vi "FlexMag - 23-03-2023.vi"() -> ()   [LabVIEW 2018] (continued)
                    n16430 = local read "abort ch3"() -> (w21515:bool)
                    n16431 = case shown="False" w21515 {
                      frame False {
                        n16432 = while {
                          i -> [w21518]
                          stop <- w21521 stop-if-true
                          n16433 = Greater Or Equal?(x=w21518, y=100) -> (x >= y?=w21519:bool)
                          n16434 = case shown="True" w21519 {
                            frame False {
                            }
                            frame True {
                              n16435 = local write "Warning Message"("CH3 PumpDown process  is canceled !\nCH3 PL VBV couldn't be closed" ("Warning Message")) -> ()
                              n16436 = local write "ch3 pumpdown error"(TRUE ("ch1 pumpdown error")) -> ()
                            }
                          }
                          n16437 = local read "CH3_PL_VBV_DI"() -> (w21516:bool)
                          n16438 = local read "ch3 pumpdown alg"() -> (w21524:bool)
                          n16439 = case shown="True" w21516 {
                            tunnel: [TRUE FALSE] -> w21520
                            frame False {
                            }
                            frame True {
                              n16440 = Wait Until Next ms Multiple(millisecond multiple=u32 200) -> ()  [unwired: 1 out]
                              n16441 = local write "CH3_PL_VBV_DO"(FALSE ("CH1_CH_VBV_DO")) -> ()
                            }
                          }
                          n16442 = local read "abort ch3"() -> (w21522:bool)
                          n16443 = Not(x=w21524) -> (.not. x?=w21523:bool)
                          n16444 = Compound Arithmetic op=OR(w21520, w21522, w21523) -> (w21521:bool)
                        }
                      }
                      frame True {
                      }
                    }
                  }
                }
              }
              frame #6 {
                n16445 = local read "ch3 pumpdown alg"() -> (w21531:bool)
                n16446 = case shown="True" w21531 {
                  frame False {
                  }
                  frame True {
                    n16447 = local read "abort ch3"() -> (w21532:bool)
                    n16448 = case shown="False" w21532 {
                      frame False {
                        n16449 = local write "ch3 pl vbv close led"(TRUE ("ch1 ch vbv close")) -> ()
                        n16450 = Wait (ms)(milliseconds to wait=u32 1000) -> ()  [unwired: 1 out]
                      }
                      frame True {
                      }
                    }
                  }
                }
              }
              frame #7 {
                n16451 = local read "ch3 pumpdown alg"() -> (w21535:bool)
                n16452 = case shown="True" w21535 {
                  frame False {
                  }
                  frame True {
                    n16453 = local read "abort ch3"() -> (w21536:bool)
                    n16454 = case shown="False" w21536 {
                      frame False {
                        n16455 = local read "ch4 ch pg torr"() -> (w21539:dbl)
                        n16456 = local read "CH3_CH_ATM_DI"() -> (w21540:bool)
                        n16457 = Less?(x=w21539, y=0.5) -> (x < y?=w21541:bool)
                        n16458 = And(x=w21540, y=w21541) -> (x .and. y?=w21537:bool)
                        n16459 = case shown="True" w21537 {
                          frame False {
                            # "ch trns bp left close"
                            n16460 = while {
                              i -> [w21544]
                              stop <- w21547 stop-if-true
                              n16461 = Greater Or Equal?(x=w21544, y=100) -> (x >= y?=w21545:bool)
                              n16462 = case shown="True" w21545 {
                                frame False {
                                }
                                frame True {
                                n16463 = local write "Warning Message"("CH3 PumpDown process  is canceled !\nCH3 TRNS BP Left couldn't be closed" ("Warning Message")) -> ()
                                n16464 = local write "ch3 pumpdown error"(TRUE ("ch1 pumpdown error")) -> ()
                                }
                              }
                              n16465 = local read "CH3_Trns_BP_Left_DI"() -> (w21542:bool)
                              n16466 = local read "ch3 pumpdown alg"() -> (w21550:bool)
                              n16467 = case shown="True" w21542 {
                                tunnel: [TRUE FALSE] -> w21546
                                frame False {
                                }
                                frame True {
                                n16468 = local write "CH3_Trns_BP_Left_DO"(FALSE ("CH1_CH_VBV_DO")) -> ()
                                n16469 = Wait Until Next ms Multiple(millisecond multiple=u32 200) -> ()  [unwired: 1 out]
                                }
                              }
                              n16470 = local read "abort ch3"() -> (w21548:bool)
                              n16471 = Not(x=w21550) -> (.not. x?=w21549:bool)
                              n16472 = Compound Arithmetic op=OR(w21546, w21548, w21549) -> (w21547:bool)
                            }
                          }
                          frame True {
                            # "ch trns bp left open"
                            n16473 = while {
                              i -> [w21559]
                              stop <- w21562 stop-if-true
                              n16474 = Greater Or Equal?(x=w21559, y=100) -> (x >= y?=w21560:bool)
                              n16475 = case shown="True" w21560 {
                                frame False {
                                }
                                frame True {
                                n16476 = local write "Warning Message"("CH3 PumpDown process  is canceled !\nCH3 TRNS BP Left couldn't be opened" ("Warning Message")) -> ()
                                n16477 = local write "ch3 pumpdown error"(TRUE ("ch1 pumpdown error")) -> ()
                                }
                              }
                              n16478 = local read "CH3_Trns_BP_Left_DI"() -> (w21557:bool)
                              n16479 = local read "ch3 pumpdown alg"() -> (w21565:bool)
                              n16480 = case shown="False" w21557 {
                                tunnel: [FALSE TRUE] -> w21561
                                frame False {
                                n16481 = local write "CH3_Trns_BP_Left_DO"(TRUE ("CH1_CH_VBV_DO")) -> ()
                                n16482 = Wait Until Next ms Multiple(millisecond multiple=u32 200) -> ()  [unwired: 1 out]
                                }
                                frame True {
                                }
                              }
                              n16483 = local read "abort ch3"() -> (w21563:bool)
                              n16484 = Not(x=w21565) -> (.not. x?=w21564:bool)
                              n16485 = Compound Arithmetic op=OR(w21561, w21563, w21564) -> (w21562:bool)
                            }
                          }
                        }
                      }
                      frame True {
                      }
                    }
                  }
                }
              }
              frame #8 {
                n16486 = local read "ch3 pumpdown alg"() -> (w21572:bool)
                n16487 = case shown="True" w21572 {
                  frame False {
                  }
                  frame True {
                    n16488 = local read "abort ch3"() -> (w21573:bool)
                    n16489 = case shown="False" w21573 {
                      frame False {
                        n16490 = local read "CH3_Trns_BP_Left_DI"() -> (w21574:bool)
                        n16491 = case shown="False" w21574 {
                          frame False {
                            n16492 = local write "ch3 trns bp left close led"(TRUE ("ch1 ch vbv close")) -> ()
                            n16493 = Wait (ms)(milliseconds to wait=u32 1000) -> ()  [unwired: 1 out]
                          }
                          frame True {
                          }
                        }
                      }
                      frame True {
                      }
                    }
                  }
                }
              }
              frame #9 {
                n16494 = local read "ch3 pumpdown alg"() -> (w21577:bool)
                n16495 = case shown="True" w21577 {
                  frame False {
                  }
                  frame True {
                    n16496 = local read "abort ch3"() -> (w21578:bool)
                    n16497 = case shown="False" w21578 {
                      frame False {
                        n16498 = local read "ch2 ch pg torr"() -> (w21581:dbl)
                        n16499 = local read "CH3_CH_ATM_DI"() -> (w21582:bool)
                        n16500 = Less?(x=w21581, y=0.5) -> (x < y?=w21583:bool)
                        n16501 = And(x=w21582, y=w21583) -> (x .and. y?=w21579:bool)
                        n16502 = case shown="False" w21579 {
                          frame False {
                            # "ch trns bp right close"
                            n16503 = while {
                              i -> [w21586]
                              stop <- w21589 stop-if-true
                              n16504 = Greater Or Equal?(x=w21586, y=100) -> (x >= y?=w21587:bool)
                              n16505 = case shown="True" w21587 {
                                frame False {
                                }
                                frame True {
                                n16506 = local write "Warning Message"("CH3 PumpDown process  is canceled !\nCH3 TRNS BP Right couldn't be closed" ("Warning Message")) -> ()
                                n16507 = local write "ch3 pumpdown error"(TRUE ("ch1 pumpdown error")) -> ()
                                }
                              }
                              n16508 = local read "CH3_Trns_BP_Right_DI"() -> (w21584:bool)
                              n16509 = local read "ch3 pumpdown alg"() -> (w21592:bool)
                              n16510 = case shown="True" w21584 {
                                tunnel: [TRUE FALSE] -> w21588
                                frame False {
                                }
                                frame True {
                                n16511 = local write "CH3_Trns_BP_Right_DO"(FALSE ("CH1_CH_VBV_DO")) -> ()
                                n16512 = Wait Until Next ms Multiple(millisecond multiple=u32 200) -> ()  [unwired: 1 out]
                                }
                              }
                              n16513 = local read "abort ch3"() -> (w21590:bool)
                              n16514 = Not(x=w21592) -> (.not. x?=w21591:bool)
                              n16515 = Compound Arithmetic op=OR(w21588, w21590, w21591) -> (w21589:bool)
                            }
                          }
                          frame True {
                            # "ch trns bp right open"
                            n16516 = while {
                              i -> [w21601]
                              stop <- w21604 stop-if-true
                              n16517 = Greater Or Equal?(x=w21601, y=100) -> (x >= y?=w21602:bool)
                              n16518 = case shown="True" w21602 {
                                frame False {
                                }
                                frame True {
                                n16519 = local write "Warning Message"("CH3 PumpDown process  is canceled !\nCH3 TRNS BP Right couldn't be opened" ("Warning Message")) -> ()
                                n16520 = local write "ch3 pumpdown error"(TRUE ("ch1 pumpdown error")) -> ()
                                }
                              }
                              n16521 = local read "CH3_Trns_BP_Right_DI"() -> (w21599:bool)
                              n16522 = local read "ch3 pumpdown alg"() -> (w21607:bool)
                              n16523 = case shown="False" w21599 {
                                tunnel: [FALSE TRUE] -> w21603
                                frame False {
                                n16524 = local write "CH3_Trns_BP_Right_DO"(TRUE ("CH1_CH_VBV_DO")) -> ()
                                n16525 = Wait Until Next ms Multiple(millisecond multiple=u32 200) -> ()  [unwired: 1 out]
                                }
                                frame True {
                                }
                              }
                              n16526 = local read "abort ch3"() -> (w21605:bool)
                              n16527 = Not(x=w21607) -> (.not. x?=w21606:bool)
                              n16528 = Compound Arithmetic op=OR(w21603, w21605, w21606) -> (w21604:bool)
                            }
                          }
                        }
                      }
                      frame True {
                      }
                    }
                  }
                }
              }
              frame #10 {
                n16529 = local read "ch3 pumpdown alg"() -> (w21614:bool)
                n16530 = case shown="True" w21614 {
                  frame False {
                  }
                  frame True {
                    n16531 = local read "abort ch3"() -> (w21615:bool)
                    n16532 = case shown="False" w21615 {
                      frame False {
                        n16533 = local read "CH3_Trns_BP_Right_DI"() -> (w21616:bool)
                        n16534 = case shown="False" w21616 {
                          frame False {
                            n16535 = local write "ch3 trns bp right close led"(TRUE ("ch1 ch vbv close")) -> ()
                            n16536 = Wait (ms)(milliseconds to wait=u32 1000) -> ()  [unwired: 1 out]
                          }
                          frame True {
                          }
                        }
                      }
                      frame True {
                      }
                    }
                  }
                }
              }
              frame #11 {
                # "ch trns gv 2-3 close"
                n16537 = local read "ch3 pumpdown alg"() -> (w21619:bool)
                n16538 = case shown="True" w21619 {
                  frame False {
                  }
                  frame True {
                    n16539 = local read "abort ch3"() -> (w21620:bool)
                    n16540 = case shown="False" w21620 {
                      frame False {
                        n16541 = while {
                          i -> [w21623]
                          stop <- w21626 stop-if-true
                          n16542 = Greater Or Equal?(x=w21623, y=100) -> (x >= y?=w21624:bool)
                          n16543 = case shown="True" w21624 {
                            frame False {
                            }
                            frame True {
                              n16544 = local write "Warning Message"("CH3 PumpDown process  is canceled !\nCH3 TRNS GV couldn't be closed" ("Warning Message")) -> ()
                              n16545 = local write "ch3 pumpdown error"(TRUE ("ch1 pumpdown error")) -> ()
                            }
                          }
                          n16546 = local read "CH2_Trns_Gv_Close_DI"() -> (w21621:bool)
                          n16547 = case shown="False" w21621 {
                            tunnel: [FALSE TRUE] -> w21625
                            frame False {
                              w21633 = TRUE ("CH1_CH_VBV_DO")
                              n16548 = Not(x=w21633) -> (.not. x?=w21632:bool)
                              n16549 = local write "CH2_Trns_GV_Open_DO"(w21632) -> ()
                              n16550 = local write "CH2_Trns_GV_Close_DO"(w21633) -> ()
                              n16551 = Wait Until Next ms Multiple(millisecond multiple=u32 200) -> ()  [unwired: 1 out]
                            }
                            frame True {
                            }
                          }
                          n16552 = local read "ch2 pumpdown alg"() -> (w21629:bool)
                          n16553 = local read "abort ch3"() -> (w21627:bool)
                          n16554 = Not(x=w21629) -> (.not. x?=w21628:bool)
                          n16555 = Compound Arithmetic op=OR(w21625, w21627, w21628) -> (w21626:bool)
                        }
                      }
                      frame True {
                      }
                    }
                  }
                }
              }
              frame #12 {
                n16556 = local read "ch3 pumpdown alg"() -> (w21637:bool)
                n16557 = case shown="True" w21637 {
                  frame False {
                  }
                  frame True {
                    n16558 = local read "abort ch3"() -> (w21638:bool)
                    n16559 = case shown="False" w21638 {
                      frame False {
                        n16560 = local write "ch3-ch2 trns gv close led"(TRUE ("ch3-ch2 gv close led")) -> ()
                        n16561 = Wait (ms)(milliseconds to wait=u32 1000) -> ()  [unwired: 1 out]
                      }
                      frame True {
                      }
                    }
                  }
                }
              }
              frame #13 {
                # "ch trns gv 3-4 close"
                n16562 = local read "ch3 pumpdown alg"() -> (w21641:bool)
                n16563 = case shown="True" w21641 {
                  frame False {
                  }
                  frame True {
                    n16564 = local read "abort ch3"() -> (w21642:bool)
                    n16565 = case shown="False" w21642 {
                      frame False {
                        n16566 = while {
                          i -> [w21645]
                          stop <- w21648 stop-if-true
                          n16567 = Greater Or Equal?(x=w21645, y=100) -> (x >= y?=w21646:bool)
                          n16568 = case shown="True" w21646 {
                            frame False {
                            }
                            frame True {
                              n16569 = local write "Warning Message"("CH3 PumpDown process  is canceled !\nCH3-CH4 TRNS GV couldn't be closed" ("Warning Message")) -> ()
                              n16570 = local write "ch3 pumpdown error"(TRUE ("ch1 pumpdown error")) -> ()
                            }
                          }
                          n16571 = local read "CH3_Trns_Gv_Close_DI"() -> (w21643:bool)
                          n16572 = case shown="False" w21643 {
                            tunnel: [FALSE TRUE] -> w21647
                            frame False {
                              n16573 = local write "CH3_Trns_GV_Open_DO"(FALSE ("CH3_Trns_GV_Open_DO")) -> ()
                              n16574 = local write "CH3_Trns_GV_Close_DO"(TRUE ("CH1_CH_VBV_DO")) -> ()
                              n16575 = Wait Until Next ms Multiple(millisecond multiple=u32 200) -> ()  [unwired: 1 out]
                            }
                            frame True {
                            }
                          }
                          n16576 = local read "ch3 pumpdown alg"() -> (w21651:bool)
                          n16577 = local read "abort ch3"() -> (w21649:bool)
                          n16578 = Not(x=w21651) -> (.not. x?=w21650:bool)
                          n16579 = Compound Arithmetic op=OR(w21647, w21649, w21650) -> (w21648:bool)
                        }
                      }
                      frame True {
                      }
                    }
                  }
                }
              }
              frame #14 {
                n16580 = local read "ch3 pumpdown alg"() -> (w21659:bool)
                n16581 = case shown="True" w21659 {
                  frame False {
                  }
                  frame True {
                    n16582 = local read "abort ch3"() -> (w21660:bool)
                    n16583 = case shown="False" w21660 {
                      frame False {
                        n16584 = local write "ch3-ch4 trns gv close led"(TRUE ("ch1 ch vbv close")) -> ()
                        n16585 = Wait (ms)(milliseconds to wait=u32 1000) -> ()  [unwired: 1 out]
                      }
                      frame True {
                      }
                    }
                  }
                }
              }
              frame #15 {
                # "tp bv open\npc gv open"
                n16586 = local read "ch3 pumpdown alg"() -> (w21663:bool)
                n16587 = case shown="True" w21663 {
                  frame False {
                  }
                  frame True {
                    n16588 = local read "abort ch3"() -> (w21664:bool)
                    n16589 = case shown="False" w21664 {
                      frame False {
                        n16590 = local read "CH3_CH_ATM_DI"() -> (w21666:bool)
                        n16591 = local read "CH3_PL_ATM_DI"() -> (w21667:bool)
                        n16592 = And(x=w21666, y=w21667) -> (x .and. y?=w21665:bool)
                        n16593 = case shown="True" w21665 {
                          frame False {
                          }
                          frame True {
                            n16594 = stacked-sequence {
                              frame #0 {
                                # "tp bv open\npc gv open"
                              }
                              frame #1 {
                                n16595 = while {
                                i -> [w21670]
                                stop <- w21673 stop-if-true
                                n16596 = Greater Or Equal?(x=w21670, y=100) -> (x >= y?=w21671:bool)
                                n16597 = case shown="True" w21671 {
                                frame False {
                                }
                                frame True {
                                n16598 = local write "Warning Message"("CH3 PumpDown process  is canceled !\nCH3 TP BV couldn't be opened" ("Warning Message")) -> ()
                                n16599 = local write "ch3 pumpdown error"(TRUE ("ch1 pumpdown error")) -> ()
                                }
                                }
                                n16600 = local read "CH3_TP_BV_DI"() -> (w21668:bool)
                                n16601 = local read "ch3 pumpdown alg"() -> (w21676:bool)
                                n16602 = case shown="False" w21668 {
                                tunnel: [FALSE TRUE] -> w21672
                                frame False {
                                n16603 = Wait Until Next ms Multiple(millisecond multiple=u32 200) -> ()  [unwired: 1 out]
                                n16604 = local write "CH3_TP_BV_DO"(TRUE ("CH1_CH_VBV_DO")) -> ()
                                }
                                frame True {
                                }
                                }
                                n16605 = local read "abort ch3"() -> (w21674:bool)
                                n16606 = Not(x=w21676) -> (.not. x?=w21675:bool)
                                n16607 = Compound Arithmetic op=OR(w21672, w21674, w21675) -> (w21673:bool)
                                }
                              }
                              frame #2 {
                                n16608 = local read "ch3 pumpdown alg"() -> (w21683:bool)
                                n16609 = case shown="True" w21683 {
                                frame False {
                                }
                                frame True {
                                n16610 = local write "ch3 tp bv open led"(TRUE ("ch1 tp bv open led")) -> ()
                                n16611 = Wait (ms)(milliseconds to wait=u32 1000) -> ()  [unwired: 1 out]
                                }
                                }
                              }
                              frame #3 {
                                n16612 = stacked-sequence {
                                frame #0 {
                                n16613 = local read "ch3 pumpdown alg"() -> (w21686:bool)
                                n16614 = case shown="True" w21686 {
                                frame False {
                                }
                                frame True {
                                n16615 = flat-sequence {
                                frame #0 {
                                n16616 = local write "pcgv3 auto open"(TRUE ("pcgv1 auto open")) -> ()
                                }
                                frame #1 {
                                n16617 = Wait (ms)(milliseconds to wait=u32 2000) -> ()  [unwired: 1 out]
                                }
                                frame #2 {
                                n16618 = local write "pcgv3 auto open"(TRUE ("pcgv1 auto open")) -> ()
                                }
                                }
                                }
                                }
                                }
                                frame #1 {
                                n16619 = while {
                                i -> [w21696]
                                stop <- w21692 stop-if-true
                                n16620 = Greater Or Equal?(x=w21696, y=200) -> (x >= y?=w21698:bool)
                                n16621 = case shown="True" w21698 {
                                frame False {
                                }
                                frame True {
                                n16622 = local write "ch3 pumpdown error"(TRUE ("ch1 pumpdown error")) -> ()
                                n16623 = local write "Warning Message"("CH3 PumpDown process  is canceled !\nCH3 PC GV couldn't be opened" ("Warning Message")) -> ()
                                }
                                }
                                n16624 = local read "ch3 pumpdown alg"() -> (w21695:bool)
                                n16625 = local read "ch3_pcgv_gui"() -> (w21691:bool)
                                n16626 = local read "abort ch3"() -> (w21693:bool)
                                n16627 = Wait Until Next ms Multiple(millisecond multiple=u32 200) -> ()  [unwired: 1 out]
                                n16628 = Not(x=w21695) -> (.not. x?=w21694:bool)
                                n16629 = Compound Arithmetic op=OR(w21691, w21693, w21694) -> (w21692:bool)
                                }
                                }
                                }
                              }
                              frame #4 {
                                n16630 = local read "ch3 pumpdown alg"() -> (w21701:bool)
                                n16631 = case shown="True" w21701 {
                                frame False {
                                }
                                frame True {
                                n16632 = local write "ch3 pc gv open led"(TRUE ("ch1 tp bv open led")) -> ()
                                n16633 = Wait (ms)(milliseconds to wait=u32 1000) -> ()  [unwired: 1 out]
                                }
                                }
                              }
                            }
                          }
                        }
                      }
                      frame True {
                      }
                    }
                  }
                }
              }
              frame #16 {
                n16634 = stacked-sequence {
                  frame #0 {
                    n16635 = local read "ch3 pumpdown alg"() -> (w21704:bool)
                    n16636 = case shown="True" w21704 {
                      frame False {
                      }
                      frame True {
                        n16637 = local read "abort ch3"() -> (w21705:bool)
                        n16638 = case shown="False" w21705 {
                          frame False {
                            n16639 = local write "CH3_PL_ATM_DO"(TRUE ("CH1_PL_ATM_DO")) -> ()
                            n16640 = Wait (ms)(milliseconds to wait=u32 2000) -> ()  [unwired: 1 out]
                          }
                          frame True {
                          }
                        }
                      }
                    }
                  }
                  frame #1 {
                    n16641 = local read "ch3 pumpdown alg"() -> (w21708:bool)
                    n16642 = case shown="True" w21708 {
                      frame False {
                      }
                      frame True {
                        n16643 = local read "abort ch3"() -> (w21709:bool)
                        n16644 = case shown="False" w21709 {
                          frame False {
                            n16645 = local write "CH3_CH_ATM_DO"(TRUE ("CH1_CH_ATM_DO")) -> ()
                            n16646 = Wait (ms)(milliseconds to wait=u32 2000) -> ()  [unwired: 1 out]
                          }
                          frame True {
                          }
                        }
                      }
                    }
                  }
                }
              }
              frame #17 {
                # "mp start"
                n16647 = local read "ch3 pumpdown alg"() -> (w21712:bool)
                n16648 = case shown="True" w21712 {
                  frame False {
                  }
                  frame True {
                    n16649 = local read "abort ch3"() -> (w21713:bool)
                    n16650 = case shown="False" w21713 {
                      frame False {
                        n16651 = while {
                          i -> [w21718]
                          stop <- w21722 stop-if-true
                          n16652 = Greater?(x=w21718, y=100) -> (0:w21714:bool)
                          n16653 = case shown="True" w21714 {
                            frame False {
                            }
                            frame True {
                              n16654 = local write "Warning Message"("CH3 PumpDown process  is canceled !\nCH3 MP couldn't be started" ("Warning Message")) -> ()
                              n16655 = local write "ch3 pumpdown error"(TRUE ("ch1 pumpdown error")) -> ()
                            }
                          }
                          n16656 = local read "CH3_MP_DI"() -> (w21716:bool)
                          n16657 = case shown="False" w21716 {
                            tunnel: [FALSE TRUE] -> w21715
                            frame False {
                              n16658 = Wait Until Next ms Multiple(millisecond multiple=u32 200) -> ()  [unwired: 1 out]
                              n16659 = local write "CH3_MP_DO"(TRUE ("CH1_MP_DO")) -> ()
                            }
                            frame True {
                            }
                          }
                          n16660 = local read "ch3 pumpdown alg"() -> (w21721:bool)
                          n16661 = local read "abort ch3"() -> (w21719:bool)
                          n16662 = Not(x=w21721) -> (.not. x?=w21720:bool)
                          n16663 = Compound Arithmetic op=OR(w21715, w21719, w21720) -> (w21722:bool)
                        }
                      }
                      frame True {
                      }
                    }
                  }
                }
              }
              frame #18 {
                n16664 = local read "ch3 pumpdown alg"() -> (w21729:bool)
                n16665 = case shown="True" w21729 {
                  frame False {
                  }
                  frame True {
                    n16666 = local read "abort ch3"() -> (w21730:bool)
                    n16667 = case shown="False" w21730 {
                      frame False {
                        n16668 = local write "ch3 mp start led"(TRUE ("ch1 ch vbv close")) -> ()
                        n16669 = Wait (ms)(milliseconds to wait=u32 1000) -> ()  [unwired: 1 out]
                      }
                      frame True {
                      }
                    }
                  }
                }
              }
              frame #19 {
                # "pl pg check"
                n16670 = local read "ch3 pumpdown alg"() -> (w21733:bool)
                n16671 = case shown="True" w21733 {
                  frame False {
                  }
                  frame True {
                    n16672 = local read "abort ch3"() -> (w21734:bool)
                    n16673 = case shown="False" w21734 {
                      frame False {
                        n16674 = while {
                          i -> [w21741]
                          stop <- w21745 stop-if-true
                          # "30 min"
                          n16675 = Greater?(x=w21741, y=9000) -> (0:w21738:bool)
                          n16676 = case shown="True" w21738 {
                            frame False {
                            }
                            frame True {
                              n16677 = local write "Warning Message"("CH3 PumpDown process  is canceled !\nCH3 PL Pressure couldn't reach under 0.05 Torr" ("Warning Message")) -> ()
                              n16678 = local write "ch3 pumpdown error"(TRUE ("ch1 pumpdown error")) -> ()
                            }
                          }
                          n16679 = local read "ch3 pl pg  torr"() -> (w21737:dbl)
                          n16680 = Less?(x=w21737, y=0.7) -> (x < y?=w21735:bool)
                          n16681 = case shown="False" w21735 {
                            tunnel: [FALSE TRUE] -> w21739
                            frame False {
                              n16682 = Wait Until Next ms Multiple(millisecond multiple=u32 200) -> ()  [unwired: 1 out]
                            }
                            frame True {
                            }
                          }
                          n16683 = local read "ch3 pumpdown alg"() -> (w21744:bool)
                          n16684 = local read "abort ch3"() -> (w21742:bool)
                          n16685 = Not(x=w21744) -> (.not. x?=w21743:bool)
                          n16686 = Compound Arithmetic op=OR(w21739, w21742, w21743) -> (w21745:bool)
                        }
                      }
                      frame True {
                      }
                    }
                  }
                }
              }
              frame #20 {
                n16687 = local read "ch3 pumpdown alg"() -> (w21751:bool)
                n16688 = case shown="True" w21751 {
                  frame False {
                  }
                  frame True {
                    n16689 = local read "abort ch3"() -> (w21752:bool)
                    n16690 = case shown="False" w21752 {
                      frame False {
                        n16691 = local write "ch3 pl press under 0.05 T led"(TRUE ("ch1 ch vbv close")) -> ()
                        n16692 = Wait (ms)(milliseconds to wait=u32 1000) -> ()  [unwired: 1 out]
                      }
                      frame True {
                      }
                    }
                  }
                }
              }
              frame #21 {
                # "tp bv open"
                n16693 = local read "ch3 pumpdown alg"() -> (w21755:bool)
                n16694 = case shown="True" w21755 {
                  frame False {
                  }
                  frame True {
                    n16695 = local read "abort ch3"() -> (w21756:bool)
                    n16696 = case shown="False" w21756 {
                      frame False {
                        n16697 = while {
                          i -> [w21761]
                          stop <- w21765 stop-if-true
                          n16698 = Greater?(x=w21761, y=100) -> (0:w21757:bool)
                          n16699 = case shown="True" w21757 {
                            frame False {
                            }
                            frame True {
                              n16700 = local write "Warning Message"("CH3 PumpDown process  is canceled !\nCH3 TP BV couldn't be opened" ("Warning Message")) -> ()
                              n16701 = local write "ch3 pumpdown error"(TRUE ("ch1 pumpdown error")) -> ()
                            }
                          }
                          n16702 = local read "CH3_TP_BV_DI"() -> (w21759:bool)
                          n16703 = case shown="False" w21759 {
                            tunnel: [FALSE TRUE] -> w21758
                            frame False {
                              n16704 = Wait Until Next ms Multiple(millisecond multiple=u32 200) -> ()  [unwired: 1 out]
                              n16705 = local write "CH3_TP_BV_DO"(TRUE ("CH1_MP_DO")) -> ()
                            }
                            frame True {
                            }
                          }
                          n16706 = local read "ch3 pumpdown alg"() -> (w21764:bool)
                          n16707 = local read "abort ch3"() -> (w21762:bool)
                          n16708 = Not(x=w21764) -> (.not. x?=w21763:bool)
                          n16709 = Compound Arithmetic op=OR(w21758, w21762, w21763) -> (w21765:bool)
                        }
                      }
                      frame True {
                      }
                    }
                  }
                }
              }
              frame #22 {
                n16710 = local read "ch3 pumpdown alg"() -> (w21772:bool)
                n16711 = case shown="True" w21772 {
                  frame False {
                  }
                  frame True {
                    n16712 = local read "abort ch3"() -> (w21773:bool)
                    n16713 = case shown="False" w21773 {
                      frame False {
                        n16714 = local write "ch3 tp bv open led"(TRUE ("ch1 ch vbv close")) -> ()
                        n16715 = Wait (ms)(milliseconds to wait=u32 1000) -> ()  [unwired: 1 out]
                      }
                      frame True {
                      }
                    }
                  }
                }
              }
              frame #23 {
                # "pc gv open"
                n16716 = local read "ch3 pumpdown alg"() -> (w21776:bool)
                n16717 = case shown="True" w21776 {
                  frame False {
                  }
                  frame True {
                    n16718 = local read "abort ch3"() -> (w21777:bool)
                    n16719 = case shown="False" w21777 {
                      frame False {
                        n16720 = stacked-sequence {
                          frame #0 {
                            n16721 = local read "ch3 pumpdown alg"() -> (w21778:bool)
                            n16722 = case shown="True" w21778 {
                              frame False {
                              }
                              frame True {
                                n16723 = flat-sequence {
                                frame #0 {
                                n16724 = local write "pcgv3 auto open"(TRUE ("pcgv1 auto open")) -> ()
                                }
                                frame #1 {
                                n16725 = Wait (ms)(milliseconds to wait=u32 2000) -> ()  [unwired: 1 out]
                                }
                                frame #2 {
                                n16726 = local write "pcgv3 auto open"(TRUE ("pcgv1 auto open")) -> ()
                                }
                                }
                              }
                            }
                          }
                          frame #1 {
                            n16727 = while {
                              i -> [w21788]
                              stop <- w21784 stop-if-true
                              n16728 = Greater Or Equal?(x=w21788, y=200) -> (x >= y?=w21790:bool)
                              n16729 = case shown="True" w21790 {
                                frame False {
                                }
                                frame True {
                                n16730 = local write "ch3 pumpdown error"(TRUE ("ch1 pumpdown error")) -> ()
                                n16731 = local write "Warning Message"("CH3 PumpDown process  is canceled !\nCH3 PC GV couldn't be opened" ("Warning Message")) -> ()
                                }
                              }
                              n16732 = local read "ch3 pumpdown alg"() -> (w21787:bool)
                              n16733 = local read "ch3_pcgv_gui"() -> (w21783:bool)
                              n16734 = local read "abort ch3"() -> (w21785:bool)
                              n16735 = Wait Until Next ms Multiple(millisecond multiple=u32 200) -> ()  [unwired: 1 out]
                              n16736 = Not(x=w21787) -> (.not. x?=w21786:bool)
                              n16737 = Compound Arithmetic op=OR(w21783, w21785, w21786) -> (w21784:bool)
                            }
                          }
                        }
                      }
                      frame True {
                      }
                    }
                  }
                }
              }
              frame #24 {
                n16738 = local read "ch3 pumpdown alg"() -> (w21793:bool)
                n16739 = case shown="True" w21793 {
                  frame False {
                  }
                  frame True {
                    n16740 = local read "abort ch3"() -> (w21794:bool)
                    n16741 = case shown="False" w21794 {
                      frame False {
                        n16742 = local write "ch3 pc gv open led"(TRUE ("ch1 ch vbv close")) -> ()
                        n16743 = Wait (ms)(milliseconds to wait=u32 1000) -> ()  [unwired: 1 out]
                      }
                      frame True {
                      }
                    }
                  }
                }
              }
              frame #25 {
                # "ch pressure check"
                n16744 = local read "ch3 pumpdown alg"() -> (w21797:bool)
                n16745 = case shown="True" w21797 {
                  frame False {
                  }
                  frame True {
                    n16746 = local read "abort ch3"() -> (w21798:bool)
                    n16747 = case shown="False" w21798 {
                      frame False {
                        n16748 = while {
                          i -> [w21805]
                          stop <- w21809 stop-if-true
                          # "30 min"
                          n16749 = Greater?(x=w21805, y=9000) -> (0:w21802:bool)
                          n16750 = case shown="True" w21802 {
                            frame False {
                            }
                            frame True {
                              n16751 = local write "Warning Message"("CH3 PumpDown process  is canceled !\nCH3 CH Pressure couldn't reach under 0.5 Torr" ("Warning Message")) -> ()
                              n16752 = local write "ch3 pumpdown alg"(TRUE ("ch1 pumpdown error")) -> ()
                            }
                          }
                          n16753 = local read "ch3 ch pg torr"() -> (w21801:dbl)
                          n16754 = Less Or Equal?(x=w21801, y=0.5) -> (x <= y?=w21799:bool)
                          n16755 = case shown="False" w21799 {
                            tunnel: [FALSE TRUE] -> w21803
                            frame False {
                              n16756 = Wait Until Next ms Multiple(millisecond multiple=u32 200) -> ()  [unwired: 1 out]
                            }
                            frame True {
                            }
                          }
                          n16757 = local read "ch3 pumpdown alg"() -> (w21808:bool)
                          n16758 = local read "abort ch3"() -> (w21806:bool)
                          n16759 = Not(x=w21808) -> (.not. x?=w21807:bool)
                          n16760 = Compound Arithmetic op=OR(w21803, w21806, w21807) -> (w21809:bool)
                        }
                      }
                      frame True {
                      }
                    }
                  }
                }
              }
              frame #26 {
                n16761 = local read "ch3 pumpdown alg"() -> (w21815:bool)
                n16762 = case shown="True" w21815 {
                  frame False {
                  }
                  frame True {
                    n16763 = local read "abort ch3"() -> (w21816:bool)
                    n16764 = case shown="False" w21816 {
                      frame False {
                        n16765 = local write "ch3 ch press under 0.5 T led"(TRUE ("ch1 ch pressure led")) -> ()
                        n16766 = Wait (ms)(milliseconds to wait=u32 1000) -> ()  [unwired: 1 out]
                      }
                      frame True {
                      }
                    }
                  }
                }
              }
              frame #27 {
                # "ch 2 pressure check\nfor trns bp bv"
                n16767 = local read "ch3 pumpdown alg"() -> (w21819:bool)
                n16768 = case shown="True" w21819 {
                  frame False {
                  }
                  frame True {
                    n16769 = local read "abort ch3"() -> (w21820:bool)
                    n16770 = case shown="False" w21820 {
                      frame False {
                        n16771 = local read "ch2 ch pg torr"() -> (w21823:dbl)
                        n16772 = Less Or Equal?(x=w21823, y=0.5) -> (x <= y?=w21821:bool)
                        n16773 = case shown="True" w21821 {
                          frame False {
                          }
                          frame True {
                            n16774 = stacked-sequence {
                              frame #0 {
                                n16775 = while {
                                i -> [w21828]
                                stop <- w21832 stop-if-true
                                n16776 = Greater?(x=w21828, y=100) -> (0:w21825:bool)
                                n16777 = case shown="True" w21825 {
                                frame False {
                                }
                                frame True {
                                n16778 = local write "ch3 pumpdown error"(TRUE ("ch1 pumpdown error")) -> ()
                                n16779 = local write "Warning Message"("CH3 PumpDown process  is canceled !\nCH3 Trns BP Right couldn't be opened" ("Warning Message")) -> ()
                                }
                                }
                                n16780 = local read "CH3_Trns_BP_Right_DI"() -> (w21824:bool)
                                n16781 = case shown="False" w21824 {
                                tunnel: [FALSE TRUE] -> w21826
                                frame False {
                                n16782 = local write "CH3_Trns_BP_Right_DO"(TRUE ("CH1_Trns_BP_Left_DO")) -> ()
                                n16783 = Wait Until Next ms Multiple(millisecond multiple=u32 200) -> ()  [unwired: 1 out]
                                }
                                frame True {
                                }
                                }
                                n16784 = local read "ch3 pumpdown alg"() -> (w21831:bool)
                                n16785 = local read "abort ch3"() -> (w21829:bool)
                                n16786 = Not(x=w21831) -> (.not. x?=w21830:bool)
                                n16787 = Compound Arithmetic op=OR(w21826, w21829, w21830) -> (w21832:bool)
                                }
                              }
                              frame #1 {
                                n16788 = local read "ch3 pumpdown alg"() -> (w21839:bool)
                                n16789 = case shown="True" w21839 {
                                frame False {
                                }
                                frame True {
                                n16790 = local read "abort ch3"() -> (w21840:bool)
                                n16791 = case shown="False" w21840 {
                                frame False {
                                n16792 = local write "ch3 trns bp right open led"(TRUE ("ch1 tp start led")) -> ()
                                n16793 = local write "ch2_3 vacuum level"("VACUUM" ("ch3_4 vacuum level")) -> ()
                                n16794 = Wait (ms)(milliseconds to wait=u32 1000) -> ()  [unwired: 1 out]
                                }
                                frame True {
                                }
                                }
                                }
                                }
                              }
                              frame #2 {
                                n16795 = while {
                                i -> [w21846]
                                stop <- w21848 stop-if-true
                                n16796 = local read "ch3 pumpdown alg"() -> (w21849:bool)
                                n16797 = Wait Until Next ms Multiple(millisecond multiple=u32 200) -> ()  [unwired: 1 out]
                                n16798 = local read "abort ch3"() -> (w21851:bool)
                                n16799 = Greater?(x=w21846, y=100) -> (0:w21845:bool)
                                n16800 = Not(x=w21849) -> (.not. x?=w21850:bool)
                                n16801 = Compound Arithmetic op=OR(w21845, w21851, w21850) -> (w21848:bool)
                                }
                              }
                            }
                          }
                        }
                      }
                      frame True {
                      }
                    }
                  }
                }
              }
              frame #28 {
              }
              frame #29 {
                # "ch 4 pressure check\nfor trns bp bv"
                n16802 = local read "ch3 pumpdown alg"() -> (w21852:bool)
                n16803 = case shown="True" w21852 {
                  frame False {
                  }
                  frame True {
                    n16804 = local read "abort ch3"() -> (w21853:bool)
                    n16805 = case shown="False" w21853 {
                      frame False {
                        n16806 = local read "ch4 ch pg torr"() -> (w21856:dbl)
                        n16807 = Less Or Equal?(x=w21856, y=0.5) -> (x <= y?=w21854:bool)
                        n16808 = case shown="True" w21854 {
                          frame False {
                          }
                          frame True {
                            n16809 = stacked-sequence {
                              frame #0 {
                                n16810 = while {
                                i -> [w21861]
                                stop <- w21865 stop-if-true
                                n16811 = Greater?(x=w21861, y=100) -> (0:w21858:bool)
                                n16812 = case shown="True" w21858 {
                                frame False {
                                }
                                frame True {
                                n16813 = local write "Warning Message"("CH3 PumpDown process  is canceled !\nCH3 Trns BP Left couldn't be opened" ("Warning Message")) -> ()
                                n16814 = local write "ch3 pumpdown error"(TRUE ("ch1 pumpdown error")) -> ()
                                }
                                }
                                n16815 = local read "CH3_Trns_BP_Left_DI"() -> (w21857:bool)
                                n16816 = case shown="False" w21857 {
                                tunnel: [FALSE TRUE] -> w21859
                                frame False {
                                n16817 = local write "CH3_Trns_BP_Left_DO"(TRUE ("CH1_Trns_BP_Left_DO")) -> ()
                                n16818 = Wait Until Next ms Multiple(millisecond multiple=u32 200) -> ()  [unwired: 1 out]
                                }
                                frame True {
                                }
                                }
                                n16819 = local read "ch3 pumpdown alg"() -> (w21864:bool)
                                n16820 = local read "abort ch3"() -> (w21862:bool)
                                n16821 = Not(x=w21864) -> (.not. x?=w21863:bool)
                                n16822 = Compound Arithmetic op=OR(w21859, w21862, w21863) -> (w21865:bool)
                                }
                              }
                              frame #1 {
                                n16823 = local read "ch3 pumpdown alg"() -> (w21872:bool)
                                n16824 = case shown="True" w21872 {
                                frame False {
                                }
                                frame True {
                                n16825 = local read "abort ch3"() -> (w21873:bool)
                                n16826 = case shown="False" w21873 {
                                frame False {
                                n16827 = local write "ch3 trns bp left open led"(TRUE ("ch1 tp start led")) -> ()
                                n16828 = local write "ch3_4 vacuum level"("VACUUM" ("ch3_4 vacuum level")) -> ()
                                n16829 = Wait (ms)(milliseconds to wait=u32 1000) -> ()  [unwired: 1 out]
                                }
                                frame True {
                                }
                                }
                                }
                                }
                              }
                              frame #2 {
                                n16830 = while {
                                i -> [w21879]
                                stop <- w21881 stop-if-true
                                n16831 = Wait Until Next ms Multiple(millisecond multiple=u32 200) -> ()  [unwired: 1 out]
                                n16832 = local read "ch1 pumpdown alg"() -> (w21882:bool)
                                n16833 = local read "abort ch1"() -> (w21884:bool)
                                n16834 = Greater?(x=w21879, y=100) -> (0:w21878:bool)
                                n16835 = Not(x=w21882) -> (.not. x?=w21883:bool)
                                n16836 = Compound Arithmetic op=OR(w21878, w21884, w21883) -> (w21881:bool)
                                }
                              }
                            }
                          }
                        }
                      }
                      frame True {
                      }
                    }
                  }
                }
              }
              frame #30 {
                # "ch pressure check"
                n16837 = local read "ch3 pumpdown alg"() -> (w21885:bool)
                n16838 = case shown="True" w21885 {
                  frame False {
                  }
                  frame True {
                    n16839 = local read "abort ch3"() -> (w21886:bool)
                    n16840 = case shown="False" w21886 {
                      frame False {
                        n16841 = while {
                          i -> [w21893]
                          stop <- w21897 stop-if-true
                          # "20 min"
                          n16842 = Greater?(x=w21893, y=6000) -> (0:w21890:bool)
                          n16843 = case shown="True" w21890 {
                            frame False {
                            }
                            frame True {
                              n16844 = local write "Warning Message"("CH3 PumpDown process  is canceled !\nCH3 CH Pressure couldn't reach under 0.2 Torr" ("Warning Message")) -> ()
                              n16845 = local write "ch3 pumpdown error"(TRUE ("ch1 pumpdown error")) -> ()
                            }
                          }
                          n16846 = local read "ch3 ch pg torr"() -> (w21889:dbl)